vi "Dresden R2R Sputter 03.02.2018 IY24.vi"() -> ()   [LabVIEW 2009] (continued)
                                }
                                frame #1 {
                                n16210 = local write "Semi"(T/1 ("Semi")) -> ()
                                n16211 = local write "Error Message"("Start up process was cancelled.\nPlease check chamber \nvacuum connections." ("Error Message")) -> ()
                                }
                                }
                                n16212 = local read "Ch1_pressure"() -> (w28102)
                                n16213 = Less?(x=w28102, y=dbl? 0.9) -> (x < y?=w28100)
                                n16214 = case shown="False" w28100 {
                                tunnel: [i16? 0 T/1] -> w28105
                                frame #0 {
                                n16215 = Wait Until Next ms Multiple(millisecond multiple=i32? 500) -> ()  [unwired: 1 out]
                                }
                                frame #1 {
                                }
                                }
                                n16216 = local read "Semi"() -> (w28104)
                                n16217 = Or(x=w28105, y=w28104) -> (x .or. y?=w28103)
                                }
                                }
                                frame #1 {
                                }
                                }
                                }
                                frame #1 {
                                n16218 = local read "Semi"() -> (w28114)
                                n16219 = case shown="False" w28114 {
                                frame #0 {
                                n16220 = local write "Ch1_PA28"(T/1 ("PA3")) -> ()
                                n16221 = Wait Until Next ms Multiple(millisecond multiple=i32? 1000) -> ()  [unwired: 1 out]
                                }
                                frame #1 {
                                }
                                }
                                }
                                }
                              }
                              frame #1 {
                              }
                            }
                          }
                          frame #24 {
                            # "START TP"
                            n16222 = local read "Semi"() -> (w28117)
                            n16223 = case shown="False" w28117 {
                              frame #0 {
                                n16224 = stacked-sequence {
                                frame #0 {
                                n16225 = local read "Semi"() -> (w28118)
                                n16226 = case shown="False" w28118 {
                                frame #0 {
                                n16227 = stacked-sequence {
                                frame #0 {
                                n16228 = local read "Semi"() -> (w28119)
                                n16229 = case shown="False" w28119 {
                                frame #0 {
                                n16230 = local write "Tp1_auto_start"(T/1 ("Tp1_auto_start")) -> ()
                                }
                                frame #1 {
                                }
                                }
                                }
                                frame #1 {
                                n16231 = local read "Semi"() -> (w28121)
                                n16232 = case shown="False" w28121 {
                                frame #0 {
                                n16233 = Wait (ms)(milliseconds to wait=i32? 1000) -> ()  [unwired: 1 out]
                                }
                                frame #1 {
                                }
                                }
                                }
                                frame #2 {
                                n16234 = local read "Semi"() -> (w28123)
                                n16235 = case shown="False" w28123 {
                                frame #0 {
                                n16236 = while {
                                i -> [w28129]
                                stop <- w28125 stop-if-true
                                n16237 = local read "TP1_working"() -> (w28127)
                                n16238 = Greater?(x=w28129, y=i32? 120) -> (0:w28128)
                                n16239 = local read "Semi"() -> (w28126)
                                n16240 = Compound Arithmetic op=OR(w28126, w28127, w28128) -> (w28125)
                                n16241 = Wait (ms)(milliseconds to wait=i32? 500) -> ()  [unwired: 1 out]
                                }
                                }
                                frame #1 {
                                }
                                }
                                }
                                frame #3 {
                                n16242 = local read "Semi"() -> (w28131)
                                n16243 = case shown="False" w28131 {
                                frame #0 {
                                n16244 = local read "TP1_working"() -> (w28132)
                                n16245 = case shown="False" w28132 {
                                frame #0 {
                                n16246 = local write "Tp1_auto_start"(T/1 ("Pc_bv1_auto_open")) -> ()
                                }
                                frame #1 {
                                }
                                }
                                }
                                frame #1 {
                                }
                                }
                                }
                                frame #4 {
                                n16247 = local read "Semi"() -> (w28134)
                                n16248 = case shown="False" w28134 {
                                frame #0 {
                                n16249 = local read "TP1_working"() -> (w28135)
                                n16250 = case shown="False" w28135 {
                                frame #0 {
                                n16251 = Wait (ms)(milliseconds to wait=i32? 1000) -> ()  [unwired: 1 out]
                                }
                                frame #1 {
                                }
                                }
                                }
                                frame #1 {
                                }
                                }
                                }
                                frame #5 {
                                n16252 = local read "Semi"() -> (w28137)
                                n16253 = case shown="False" w28137 {
                                frame #0 {
                                n16254 = while {
                                i -> [w28143]
                                stop <- w28139 stop-if-true
                                n16255 = local read "TP1_working"() -> (w28141)
                                n16256 = Greater?(x=w28143, y=i32? 120) -> (0:w28142)
                                n16257 = local read "Semi"() -> (w28140)
                                n16258 = Compound Arithmetic op=OR(w28140, w28141, w28142) -> (w28139)
                                n16259 = Wait (ms)(milliseconds to wait=i32? 500) -> ()  [unwired: 1 out]
                                }
                                }
                                frame #1 {
                                }
                                }
                                }
                                frame #6 {
                                n16260 = local read "Semi"() -> (w28145)
                                n16261 = case shown="False" w28145 {
                                frame #0 {
                                n16262 = local read "TP1_working"() -> (w28146)
                                n16263 = case shown="False" w28146 {
                                frame #0 {
                                n16264 = local write "Error Message"("Start up process  cancelled\nbecause  TP not started.\nPlease check TP1 connections." ("Error Message")) -> ()
                                n16265 = Wait (ms)(milliseconds to wait=i32? 1000) -> ()  [unwired: 1 out]
                                }
                                frame #1 {
                                }
                                }
                                }
                                frame #1 {
                                }
                                }
                                }
                                }
                                }
                                frame #1 {
                                }
                                }
                                }
                                frame #1 {
                                n16266 = local read "Semi"() -> (w28149)
                                n16267 = case shown="False" w28149 {
                                frame #0 {
                                n16268 = local write "Ch1_PA29"(T/1 ("PA3")) -> ()
                                n16269 = Wait Until Next ms Multiple(millisecond multiple=i32? 1000) -> ()  [unwired: 1 out]
                                }
                                frame #1 {
                                }
                                }
                                }
                                }
                              }
                              frame #1 {
                              }
                            }
                          }
                          frame #25 {
                            # "CHECK CH-PRESSURE"
                            n16270 = local read "Semi"() -> (w28152)
                            n16271 = case shown="False" w28152 {
                              frame #0 {
                                n16272 = stacked-sequence {
                                frame #0 {
                                n16273 = local read "Semi"() -> (w28153)
                                n16274 = case shown="False" w28153 {
                                frame #0 {
                                n16275 = while {
                                i -> [w28162]
                                stop <- w28157 stop-if-true
                                n16276 = Greater?(x=w28162, y=i32? 240) -> (0:w28160)
                                n16277 = case shown="True" w28160 {
                                frame #0 {
                                }
                                frame #1 {
                                n16278 = local write "Semi"(T/1 ("Semi")) -> ()
                                n16279 = local write "Error Message"("Start up process was cancelled.\nPlease check chamber \nvacuum connections." ("Error Message")) -> ()
                                }
                                }
                                n16280 = local read "Ch1_pressure"() -> (w28156)
                                n16281 = Less?(x=w28156, y=dbl? 0.9) -> (x < y?=w28154)
                                n16282 = case shown="False" w28154 {
                                tunnel: [i16? 0 T/1] -> w28159
                                frame #0 {
                                n16283 = Wait Until Next ms Multiple(millisecond multiple=i32? 500) -> ()  [unwired: 1 out]
                                }
                                frame #1 {
                                }
                                }
                                n16284 = local read "Semi"() -> (w28158)
                                n16285 = Or(x=w28159, y=w28158) -> (x .or. y?=w28157)
                                }
                                }
                                frame #1 {
                                }
                                }
                                }
                                frame #1 {
                                n16286 = local read "Semi"() -> (w28168)
                                n16287 = case shown="False" w28168 {
                                frame #0 {
                                n16288 = local write "Ch1_PA30"(T/1 ("PA3")) -> ()
                                n16289 = Wait Until Next ms Multiple(millisecond multiple=i32? 1000) -> ()  [unwired: 1 out]
                                }
                                frame #1 {
                                }
                                }
                                }
                                }
                              }
                              frame #1 {
                              }
                            }
                          }
                        }
                      }
                      frame #1 {
                      }
                    }
                  }
                }
              }
              frame #1 {
              }
            }
          }
          frame #2 {
            # "ROUTINE CHECK"
            n16290 = local read "Semi"() -> (w28171)
            n16291 = case shown="False" w28171 {
              frame #0 {
                n16292 = stacked-sequence {
                  frame #0 {
                    n16293 = local read "Semi"() -> (w28172)
                    n16294 = case shown="False" w28172 {
                      frame #0 {
                        n16295 = stacked-sequence {
                          frame #0 {
                            n16296 = local read "Semi"() -> (w28173)
                            n16297 = case shown="False" w28173 {
                              frame #0 {
                                n16298 = while {
                                i -> [w28182]
                                stop <- w28177 stop-if-true
                                n16299 = Greater?(x=w28182, y=i32? 400) -> (0:w28180)
                                n16300 = case shown="True" w28180 {
                                frame #0 {
                                }
                                frame #1 {
                                n16301 = local write "Error Message"("Start up process was cancelled.\nPlease check Chamber \nvacuum connections." ("Error Message")) -> ()
                                n16302 = local write "Semi"(T/1 ("Semi")) -> ()
                                }
                                }
                                n16303 = local read "Ch1_pressure 2"() -> (w28174)
                                n16304 = Less?(x=w28174, y=dbl? 0.01) -> (x < y?=w28175)
                                n16305 = case shown="False" w28175 {
                                tunnel: [T/1 i16? 0] -> w28179
                                frame #0 {
                                }
                                frame #1 {
                                n16306 = Wait Until Next ms Multiple(millisecond multiple=i32? 500) -> ()  [unwired: 1 out]
                                }
                                }
                                n16307 = local read "Semi"() -> (w28178)
                                n16308 = Or(x=w28179, y=w28178) -> (x .or. y?=w28177)
                                }
                              }
                              frame #1 {
                              }
                            }
                          }
                          frame #1 {
                            n16309 = local read "Semi"() -> (w28188)
                            n16310 = case shown="False" w28188 {
                              frame #0 {
                                n16311 = Wait Until Next ms Multiple(millisecond multiple=i32? 1000) -> ()  [unwired: 1 out]
                              }
                              frame #1 {
                              }
                            }
                          }
                        }
                      }
                      frame #1 {
                      }
                    }
                  }
                  frame #1 {
                    n16312 = local read "Semi"() -> (w28190)
                    n16313 = case shown="False" w28190 {
                      frame #0 {
                        n16314 = stacked-sequence {
                          frame #0 {
                            n16315 = local read "Semi"() -> (w28191)
                            n16316 = case shown="False" w28191 {
                              frame #0 {
                                n16317 = while {
                                i -> [w28198]
                                stop <- w28192 stop-if-true
                                n16318 = Greater?(x=w28198, y=i32? 80) -> (0:w28196)
                                n16319 = case shown="True" w28196 {
                                frame #0 {
                                }
                                frame #1 {
                                n16320 = local write "Semi"(T/1 ("Semi")) -> ()
                                n16321 = local write "Error Message"("Start up process  cancelled\nbecause  CC not opened.\nPlease check CH1-CC connections." ("Error Message")) -> ()
                                }
                                }
                                n16322 = local read "Ch1_Cc_on_off_di"() -> (w28195)
                                n16323 = case shown="False" w28195 {
                                tunnel: [T/1 i16? 0] -> w28194
                                frame #0 {
                                }
                                frame #1 {
                                n16324 = Wait Until Next ms Multiple(millisecond multiple=i32? 200) -> ()  [unwired: 1 out]
                                n16325 = local write "Ch1_Cc_on_off_do"(T/1 ("Ch1_Tp_bv_do")) -> ()
                                }
                                }
                                n16326 = local read "Semi"() -> (w28193)
                                n16327 = Or(x=w28194, y=w28193) -> (x .or. y?=w28192)
                                }
                              }
                              frame #1 {
                              }
                            }
                          }
                          frame #1 {
                            n16328 = local read "Semi"() -> (w28205)
                            n16329 = case shown="False" w28205 {
                              frame #0 {
                                n16330 = while {
                                i -> [w28209]
                                stop <- w28206 stop-if-true
                                n16331 = Greater Or Equal?(x=w28209, y=i32? 150) -> (x >= y?=w28207)
                                n16332 = Wait (ms)(milliseconds to wait=i32? 200) -> ()  [unwired: 1 out]
                                n16333 = local read "Semi"() -> (w28211)
                                n16334 = Compound Arithmetic op=OR(w28207, w28211) -> (w28206)
                                }
                              }
                              frame #1 {
                              }
                            }
                          }
                          frame #2 {
                            n16335 = local read "Semi"() -> (w28212)
                            n16336 = case shown="False" w28212 {
                              frame #0 {
                                n16337 = local write "Ch1_PV20"(T/1 ("P1")) -> ()
                                n16338 = local write "Ch1_PA31"(T/1 ("P1")) -> ()
                                n16339 = Wait Until Next ms Multiple(millisecond multiple=i32? 2000) -> ()  [unwired: 1 out]
                              }
                              frame #1 {
                              }
                            }
                          }
                        }
                      }
                      frame #1 {
                      }
                    }
                  }
                  frame #2 {
                    n16340 = local read "Semi"() -> (w28216)
                    n16341 = case shown="False" w28216 {
                      frame #0 {
                        n16342 = stacked-sequence {
                          frame #0 {
                            n16343 = local read "Semi"() -> (w28217)
                            n16344 = case shown="False" w28217 {
                              frame #0 {
                                n16345 = while {
                                i -> [w28224]
                                stop <- w28218 stop-if-true
                                n16346 = Greater?(x=w28224, y=i32? 80) -> (0:w28222)
                                n16347 = case shown="True" w28222 {
                                frame #0 {
                                }
                                frame #1 {
                                n16348 = local write "Semi"(T/1 ("Semi")) -> ()
                                n16349 = local write "Error Message"("Start up process  cancelled\nbecause  CH1-TRNS-GV-BP2\n not opened.\nPlease check CH1-TRNS-GV-BP2\n connections." ("Error Message")) -> ()
                                }
                                }
                                n16350 = local read "Ch1_Trns_gv_bp2_di"() -> (w28221)
                                n16351 = case shown="True" w28221 {
                                tunnel: [i16? 0 T/1] -> w28220
                                frame #0 {
                                n16352 = local write "Ch1_Trns_gv_bp2_do"(i16? 0 ("Ch1_Tp_bv_do")) -> ()
                                n16353 = Wait Until Next ms Multiple(millisecond multiple=i32? 200) -> ()  [unwired: 1 out]
                                }
                                frame #1 {
                                }
                                }
                                n16354 = local read "Semi"() -> (w28219)
                                n16355 = Or(x=w28220, y=w28219) -> (x .or. y?=w28218)
                                }
                              }
                              frame #1 {
                              }
                            }
                          }
                          frame #1 {
                            n16356 = local read "Semi"() -> (w28231)
                            n16357 = case shown="False" w28231 {
                              frame #0 {
                                n16358 = local write "Ch1_PV21"(T/1 ("P1")) -> ()
                                n16359 = local write "Ch1_PA32"(T/1 ("P1")) -> ()
                                n16360 = Wait Until Next ms Multiple(millisecond multiple=i32? 2000) -> ()  [unwired: 1 out]
                              }
                              frame #1 {
                              }
                            }
                          }
                        }
                      }
                      frame #1 {
                      }
                    }
                  }
                  frame #3 {
                    n16361 = local read "Semi"() -> (w28235)
                    n16362 = case shown="False" w28235 {
                      frame #0 {
                        n16363 = stacked-sequence {
                          frame #0 {
                            n16364 = local read "Semi"() -> (w28236)
                            n16365 = case shown="False" w28236 {
                              frame #0 {
                                n16366 = while {
                                i -> [w28245]
                                stop <- w28240 stop-if-true
                                n16367 = local read "Target_time_ch1"() -> (w28239)
                                n16368 = Multiply(x=w28239, y=i32? 7200) -> (x*y=w28237)
                                n16369 = Greater?(x=w28245, y=w28237) -> (0:w28244)
                                n16370 = case shown="True" w28244 {
                                frame #0 {
                                }
                                frame #1 {
                                n16371 = local write "Semi"(T/1 ("Semi")) -> ()
                                }
                                }
                                n16372 = local read "Semi"() -> (w28243)
                                n16373 = case shown="False" w28243 {
                                tunnel: [T/1 w28250] -> w28242
                                frame #0 {
                                }
                                frame #1 {
                                n16374 = local read "Target Pressure_ch1"() -> (w28249)
                                n16375 = local read "Ch1_pressure 2"() -> (w28248)
                                n16376 = Less Or Equal?(x=w28249, y=w28248) -> (x <= y?=w28247)
                                n16377 = case shown="True" w28247 {
                                tunnel: [T/1 i16? 0] -> w28250
                                frame #0 {
                                }
                                frame #1 {
                                n16378 = Wait Until Next ms Multiple(millisecond multiple=i32? 750) -> ()  [unwired: 1 out]
                                }
                                }
                                }
                                }
                                n16379 = local read "Semi"() -> (w28241)
                                n16380 = Or(x=w28242, y=w28241) -> (x .or. y?=w28240)
                                }
                              }
                              frame #1 {
                              }
                            }
                          }
                          frame #1 {
                            n16381 = local read "Semi"() -> (w28255)
                            n16382 = case shown="False" w28255 {
                              frame #0 {
                                n16383 = Wait (ms)(milliseconds to wait=i32? 1000) -> ()  [unwired: 1 out]
                              }
                              frame #1 {
                              }
                            }
                          }
                          frame #2 {
                            n16384 = local read "Semi"() -> (w28257)
                            n16385 = case shown="False" w28257 {
                              frame #0 {
                                n16386 = local write "Ch1_PV22"(T/1 ("P1")) -> ()
                                n16387 = local write "Ch1_PA33"(T/1 ("P1")) -> ()
                                n16388 = Wait Until Next ms Multiple(millisecond multiple=i32? 1000) -> ()  [unwired: 1 out]
                              }
                              frame #1 {
                              }
                            }
                          }
                        }
                      }
                      frame #1 {
                      }
                    }
                  }
                }
              }
              frame #1 {
              }
            }
          }
          frame #3 {
            # "ROUTINE CHECK"
            n16389 = local read "Semi"() -> (w28261)
            n16390 = case shown="False" w28261 {
              frame #0 {
                n16391 = stacked-sequence {
                  frame #0 {
                    n16392 = local read "Semi"() -> (w28262)
                    n16393 = case shown="False" w28262 {
                      frame #0 {
                        w28263 = T/1 ("Visible")
                        n16394 = local write "system_status"("Start up was completed." ("system_status")) -> ()
                        n16395 = property on="final_mes_tab" class="TabCtl (strict)"("Visible"=w28263) -> ()  [unwired: 2 in, 2 out]
                        n16396 = local write "Cnt_Do_Buzzer"(w28263) -> ()
                        n16397 = Wait (ms)(milliseconds to wait=i32? 3000 ("millisecond multiple")) -> ()  [unwired: 1 out]
                      }
                      frame #1 {
                      }
                    }
                  }
                  frame #1 {
                    n16398 = local read "Semi"() -> (w28266)
                    n16399 = case shown="False" w28266 {
                      frame #0 {
                        w28268 = i16? 0 ("Visible")
                        n16400 = local write "system_status"(data[5B] ("system_status")) -> ()
                        n16401 = property on="final_mes_tab" class="TabCtl (strict)"("Visible"=w28268) -> ()  [unwired: 2 in, 2 out]
                        n16402 = local write "Start_up_ch1"(w28268) -> ()
                        n16403 = local write "Cnt_Do_Buzzer"(w28268) -> ()
                        n16404 = Wait (ms)(milliseconds to wait=i32? 3000 ("millisecond multiple")) -> ()  [unwired: 1 out]
                      }
                      frame #1 {
                      }
                    }
                  }
                  frame #2 {
                    n16405 = local read "Semi"() -> (w28270)
                    n16406 = case shown="False" w28270 {
                      frame #0 {
                        n16407 = stacked-sequence {
                          frame #0 {
                            n16408 = local write "Pps_code_entry"("PF331=" ("system_status")) -> ()
                          }
                          frame #1 {
                            n16409 = Wait (ms)(milliseconds to wait=i32? 500) -> ()  [unwired: 1 out]
                          }
                          frame #2 {
                            n16410 = local write "Ppsok"(T/1 ("Ppsok")) -> ()
                          }
                          frame #3 {
                            n16411 = Wait (ms)(milliseconds to wait=i32? 1000) -> ()  [unwired: 1 out]
                          }
                        }
                      }
                      frame #1 {
                      }
                    }
                  }
                  frame #3 {
                    n16412 = local read "Semi"() -> (w28275)
                    n16413 = case shown="False" w28275 {
                      frame #0 {
                        n16414 = stacked-sequence {
                          frame #0 {
                            n16415 = local write "Pps_code_entry"("PF227=" ("system_status")) -> ()
                          }
                          frame #1 {
                            n16416 = Wait (ms)(milliseconds to wait=i32? 500) -> ()  [unwired: 1 out]
                          }
                          frame #2 {
                            n16417 = local write "Ppsok"(T/1 ("Ppsok")) -> ()
                          }
                          frame #3 {
                            n16418 = Wait (ms)(milliseconds to wait=i32? 1000) -> ()  [unwired: 1 out]
                          }
                        }
                      }
                      frame #1 {
                      }
                    }
                  }
                  frame #4 {
                    n16419 = local read "Semi"() -> (w28280)
                    n16420 = case shown="False" w28280 {
                      frame #0 {
                        n16421 = stacked-sequence {
                          frame #0 {
                            n16422 = local write "Pps_code_entry"("PF330=" ("system_status")) -> ()
                          }
                          frame #1 {
                            n16423 = Wait (ms)(milliseconds to wait=i32? 500) -> ()  [unwired: 1 out]
                          }
                          frame #2 {
                            n16424 = local write "Ppsok"(T/1 ("Ppsok")) -> ()
                          }
                          frame #3 {
                            n16425 = Wait (ms)(milliseconds to wait=i32? 1000) -> ()  [unwired: 1 out]
                          }
                        }
                      }
                      frame #1 {
                      }
                    }
                  }
                  frame #5 {
                    n16426 = local read "Semi"() -> (w28285)
                    n16427 = case shown="False" w28285 {
                      frame #0 {
                        w28286 = T/1 ("P018")
                        n16428 = local write "Ch1_PV23"(w28286) -> ()
                        n16429 = local write "Ch1_PA34"(w28286) -> ()
                        n16430 = Wait (ms)(milliseconds to wait=i32? 1000) -> ()  [unwired: 1 out]
                      }
                      frame #1 {
                      }
                    }
                  }
                }
              }
              frame #1 {
              }
            }
          }
        }
      }
    }
    n16431 = case shown="True" "Shutdown_ch1" {
      frame #0 {
      }
      frame #1 {
        n16432 = local read "Semi"() -> (w26713:bool)
        n16433 = case shown="False" w26713 {
          frame #0 {
            n16434 = stacked-sequence {
              frame #0 {
                n16435 = local read "Semi"() -> (w26714:bool)
                n16436 = case shown="False" w26714 {
                  frame #0 {
                    n16437 = stacked-sequence {
                      frame #0 {
                        w26717 = FALSE
                        n16438 = local write "final_process_messages"("Shut Down process was completed." ("final_process_messages")) -> ()
                        n16439 = local write "system_status"("Shutting Down the System" ("system_status")) -> ()
                        n16440 = local write "Clean_shutdown_ch1"(TRUE) -> ()
                        n16441 = Wait (ms)(milliseconds to wait=u32 1000) -> ()  [unwired: 1 out]
                        "Yes" <- w26717
                        "No" <- w26717
                        "Cancel" <- w26717
                        "Close" <- w26717
                      }
                      frame #1 {
                        n16442 = call <vilib>:"Three Button Dialog.vi"("Right Button Text (\"Cancel\")"="Cancel" ("Right Button Text (\"Cancel\")"), "Center Button Text (\"No\")"="No" ("Center Button Text (\"No\")"), "Left Button Text (\"Yes\")"="Yes" ("Left Button Text (\"Yes\")"), "message"=" VENT the CHAMBER  \nLOAD or UNLOAD the substrate ? ") -> ("Which Button?"=w26723:T40)  [unwired: 7 in]
                        n16443 = case shown="\"Window Close\"" w26723 {
                          frame #0 {
                            n16444 = local write "Yes"(TRUE ("Close")) -> ()
                          }
                          frame #1 {
                            n16445 = local write "Close"(TRUE ("Close")) -> ()
                          }
                          frame #2 {
                            n16446 = local write "Cancel"(TRUE ("No")) -> ()
                          }
                          frame #3 {
                            n16447 = local write "No"(TRUE ("No")) -> ()
                          }
                        }
                      }
                      frame #2 {
                        n16448 = local read "Semi"() -> (w26729:bool)
                        n16449 = case shown="False" w26729 {
                          frame #0 {
                            n16450 = stacked-sequence {
                              frame #0 {
                                n16451 = local write "Error Message"("" ("Error Message")) -> ()
                              }
                              frame #1 {
                                n16452 = Wait (ms)(milliseconds to wait=u32 500) -> ()  [unwired: 1 out]
                              }
                              frame #2 {
                                n16453 = local write "Ppsok"(TRUE ("Ppsok")) -> ()
                              }
                              frame #3 {
                                n16454 = Wait (ms)(milliseconds to wait=u32 500) -> ()  [unwired: 1 out]
                              }
                            }
                          }
                          frame #1 {
                          }
                        }
                      }
                    }
                  }
                  frame #1 {
                  }
                }
              }
              frame #1 {
                n16455 = local read "Semi"() -> (w26734:bool)
                n16456 = case shown="False" w26734 {
                  frame #0 {
                    n16457 = local read "Cancel"() -> (w26736:bool)
                    n16458 = local read "Close"() -> (w26737:bool)
                    n16459 = Not Or(1:w26736, 2:w26737) -> (0:w26735:bool)
                    n16460 = case shown="True" w26735 {
                      frame #0 {
                        n16461 = local read "Semi"() -> (w26738:bool)
                        n16462 = case shown="False" w26738 {
                          frame #0 {
                          }
                          frame #1 {
                            n16463 = local write "Shutdown_ch1"(FALSE ("Shutdown_ch1")) -> ()
                            n16464 = local write "system_status"("Shutdown Process was completed." ("system_status")) -> ()
                          }
                        }
                      }
                      frame #1 {
                        n16465 = local read "Yes"() -> (w26743:bool)
                        n16466 = local read "No"() -> (w26742:bool)
                        n16467 = Or(x=w26743, y=w26742) -> (x .or. y?=w26741:bool)
                        n16468 = case shown="True" w26741 {
                          frame #0 {
                          }
                          frame #1 {
                            n16469 = stacked-sequence {
                              frame #0 {
                                # "CLOSE & ZERO ROUTINES"
                                n16470 = local read "Semi"() -> (w26744:bool)
                                n16471 = case shown="False" w26744 {
                                frame #0 {
                                n16472 = stacked-sequence {
                                frame #0 {
                                n16473 = local read "Semi"() -> (w26745:bool)
                                n16474 = case shown="False" w26745 {
                                frame #0 {
                                n16475 = local write "Dc_auto_off"(TRUE ("Dc_auto_off")) -> ()
                                n16476 = local write "system_status"("Shut Down in Progress for Chamber 1" ("system_status")) -> ()
                                n16477 = local write "final_process_messages"("Shut Down Process was completed for  Chamber 1." ("final_process_messages")) -> ()
                                n16478 = local write "Ch1_Sov_Ar_do"(FALSE ("Dc_auto_off")) -> ()
                                }
                                frame #1 {
                                }
                                }
                                }
                                frame #1 {
                                n16479 = local read "Semi"() -> (w26750:bool)
                                n16480 = case shown="False" w26750 {
                                frame #0 {
                                n16481 = Wait (ms)(milliseconds to wait=u32 2500) -> ()  [unwired: 1 out]
                                }
                                frame #1 {
                                }
                                }
                                }
                                frame #2 {
                                n16482 = local read "Semi"() -> (w26752:bool)
                                n16483 = case shown="False" w26752 {
                                frame #0 {
                                n16484 = local write "Ch1_Sov_Ar_do"(FALSE ("Ch1_Sov_Ar_do")) -> ()
                                n16485 = Wait (ms)(milliseconds to wait=u32 2500) -> ()  [unwired: 1 out]
                                n16486 = local write "RF_auto_off"(TRUE ("RF_auto_off")) -> ()
                                }
                                frame #1 {
                                }
                                }
                                }
                                frame #3 {
                                n16487 = local read "Semi"() -> (w26756:bool)
                                n16488 = case shown="False" w26756 {
                                frame #0 {
                                n16489 = Wait (ms)(milliseconds to wait=u32 1000) -> ()  [unwired: 1 out]
                                }
                                frame #1 {
                                }
                                }
                                }
                                }
                                }
                                frame #1 {
                                }
                                }
                              }
                              frame #1 {
                                # "STOP TP"
                                n16490 = local read "Semi"() -> (w26758:bool)
                                n16491 = case shown="False" w26758 {
                                frame #0 {
                                n16492 = stacked-sequence {
                                frame #0 {
                                n16493 = local read "Semi"() -> (w26759:bool)
                                n16494 = case shown="False" w26759 {
                                frame #0 {
                                n16495 = stacked-sequence {
                                frame #0 {
                                n16496 = local read "Semi"() -> (w26760:bool)
                                n16497 = case shown="False" w26760 {
                                frame #0 {
                                n16498 = local write "Tp1_auto_stop"(TRUE ("Tp1_auto_start")) -> ()
                                }
                                frame #1 {
                                }
                                }
                                }
                                frame #1 {
                                n16499 = local read "Semi"() -> (w26762:bool)
                                n16500 = case shown="False" w26762 {
                                frame #0 {
                                n16501 = Wait (ms)(milliseconds to wait=u32 1000) -> ()  [unwired: 1 out]
                                }
                                frame #1 {
                                }
                                }
                                }
                                frame #2 {
                                n16502 = local read "Semi"() -> (w26764:bool)
                                n16503 = case shown="False" w26764 {
                                frame #0 {
                                n16504 = while {
                                i -> [w26770]
                                stop <- w26766 stop-if-true
                                n16505 = local read "Tp1_stopped"() -> (w26768:bool)
                                n16506 = Greater?(x=w26770, y=120) -> (0:w26769:bool)
                                n16507 = local read "Semi"() -> (w26767:bool)
                                n16508 = Compound Arithmetic op=OR(w26767, w26768, w26769) -> (w26766:bool)
                                n16509 = Wait (ms)(milliseconds to wait=u32 500) -> ()  [unwired: 1 out]
                                }
                                }
                                frame #1 {
                                }
                                }
                                }
                                frame #3 {
                                n16510 = local read "Semi"() -> (w26772:bool)
                                n16511 = case shown="False" w26772 {
                                frame #0 {
                                n16512 = local read "Tp1_stopped"() -> (w26773:bool)
                                n16513 = case shown="False" w26773 {
                                frame #0 {
                                n16514 = local write "Tp1_auto_stop"(TRUE ("Pc_bv1_auto_open")) -> ()
                                }
                                frame #1 {
                                }
                                }
                                }
                                frame #1 {
                                }
                                }
                                }
                                frame #4 {
                                n16515 = local read "Semi"() -> (w26775:bool)
                                n16516 = case shown="False" w26775 {
                                frame #0 {
                                n16517 = local read "Tp1_stopped"() -> (w26776:bool)
                                n16518 = case shown="False" w26776 {
                                frame #0 {
                                n16519 = Wait (ms)(milliseconds to wait=u32 1000) -> ()  [unwired: 1 out]
                                }
                                frame #1 {